vi "pharmaBot_v0.019.vi"() -> ()   [LabVIEW 2015] (continued)
    tunnel: [w833] -> w396
    tunnel: w394 -> [w832]
    tunnel: w392 -> [_]
    tunnel: w270 -> [w826]
    tunnel: w272 -> [w825]
    tunnel: w378 -> [w824]
    tunnel: w338 -> [w823]
    shift-right: [w784] -> _
    shift-left: user_message_v6."Initializing..." ("P1 state") -> [w783]
    tunnel: w337 -> [w781]
    tunnel: w245 -> [w780]
    tunnel: w246 -> [w779]
    tunnel: [w778] -> _
    stop <- w835 stop-if-true
    # "Jumper Positions"
    # "Pipette 1 state"
    # "Add the reserved cell index from each manip when checking to see if a cell index can be added back to the queue."
    # "transform cluster + actuator"
    # "positions"
    # "Update the patched cell value visible to the user in the config menu when adding cells back into the array"
    # "If the next or previous button exceeds the index size of the patched cell indicies variable, then disable the corresponding button."
    # "Constantly check to see if there are any \ncells that have been marked as \"patched\""
    n667 = local read "Calibration Protocol"() -> (w787:T7)
    n668 = Wait (ms)(milliseconds to wait=u32 100) -> ()  [unwired: 1 out]
    n669 = local read "P1 state"() -> (w782:T11)
    n670 = local read "Patched Cell Indicies"() -> (w812:i32[])
    n671 = local read "Patched Cell Index"() -> (w811:dbl)
    n672 = local read "cells (image px)"() -> (w822:dbl[][])
    n673 = local read "Patched Cell Index"() -> (w807:dbl)
    n674 = local read "Calibrate:"() -> (w829:T8)
    n675 = local read "current cell 1"() -> (w797:i32)
    n676 = local read "unpatched cell indices"() -> (w798:i32[])
    n677 = Array Size(array=w812) -> (size(s)=w800:i32)
    n678 = Array Size(array=w822) -> (size(s)=w819:i32[])
    n679 = Increment(x=w811) -> (x+1=w810:dbl)
    n680 = Decrement(x=w807) -> (x-1=w805:dbl)
    n681 = Decrement(x=w800) -> (x-1=w799:i32)
    n682 = Index Array(array=w819, index=1) -> (element=w814:i32)
    n683 = Search 1D Array(1D array=w798, element=w797) -> (index of element=w796:i32)  [unwired: 1 in]
    n684 = Greater?(x=w810, y=w799) -> (0:w808:bool)
    n685 = Less?(x=w805, y=0.0) -> (x < y?=w806:bool)
    n686 = case shown="True" w808 {
      tunnel: [T56."Enabled" ("Disabled") T56."Disabled and Grayed Out" ("Disabled")] -> w809
      frame False {
      }
      frame True {
      }
    }
    n687 = case shown="True" w806 {
      tunnel: [T56."Enabled" ("Disabled") T56."Disabled and Grayed Out" ("Disabled")] -> w803
      frame False {
      }
      frame True {
      }
    }
    n688 = Less?(x=w796, y=0) -> (x < y?=w794:bool)
    n689 = case shown="\"manipulator 1\", Default" w829 {
      tunnel: [w854 w856 w858 w860] -> w776
      tunnel: ["Manip 1:" "Manip 2:" "Manip 3:" "Manip 4:"] -> w775
      frame "manipulator 1", Default {
        n690 = local read "current manip 1 pos (steps)"() -> (w854:i32[])
      }
      frame "manipulator 2" {
        n691 = local read "current manip 2 pos (steps)"() -> (w856:i32[])
      }
      frame "manipulator 3" {
        n692 = local read "current manip 3 pos (steps)"() -> (w858:i32[])
      }
      frame "manipulator 4" {
        n693 = local read "current manip 4 pos (steps)"() -> (w860:i32[])
      }
    }
    n694 = for {
      N: w814 -> [_]
      shift-right: [w850] -> w815
      shift-left: i32[] [] ("manip 1 cell indices 2") -> [w852]
      i -> [w851]
      n695 = Build Array (concatenate)(w852, w851) -> (w850:i32[])
    }
    n696 = case shown="True" w794 {
      tunnel: w798 -> [w840 w843]
      tunnel: [w840 w842] -> w793
      tunnel: w797 -> [_ w841]
      frame False {
      }
      frame True {
        n697 = Build Array (concatenate)(w843, w841) -> (w842:i32[])
      }
    }
    n698 = local read "current cell 2"() -> (w792:i32)
    n699 = Search 1D Array(1D array=w793, element=w792) -> (index of element=w791:i32)  [unwired: 1 in]
    n700 = Less?(x=w791, y=0) -> (x < y?=w789:bool)
    n701 = case shown="True" w789 {
      tunnel: w793 -> [w836 w839]
      tunnel: [w836 w838] -> w774
      tunnel: w792 -> [_ w837]
      frame False {
      }
      frame True {
        n702 = Build Array (concatenate)(w839, w837) -> (w838:i32[])
      }
    }
    n703 = case shown="\"Finish\"" w787 {
      tunnel: [w863 w878 w894 w919 w972 w980 w992 w1052 w1095 w1106 w1125 w1228 w1313 w1319 w1350] -> w830
      tunnel: w787 -> [w863 w877 w893 w920 w971 w979 w991 w1051 w1094 w1105 w1125 w1227 w1312 w1319 w1349]
      tunnel: [_ _ w891 _ _ _ _ _ w1093 w1104 _ _ _ _ _] -> _
      tunnel: [_ _ w891 _ _ _ _ _ w1093 w1104 _ _ _ _ _] -> _
      tunnel: [_ TRUE ("Visible") w891 w909 w969 w977 w990 w1050 w1093 w1104 _ w1225 TRUE ("Visible") _ TRUE ("Visible")] -> w827
      tunnel: [_ _ w891 w909 w969 w977 w990 w1050 w1093 w1104 _ w1225 _ _ _] -> w828
      tunnel: w826 -> [_ _ _ _ _ _ w988 w1046 w1090 w1101 _ w1222 _ _ _]
      tunnel: w825 -> [_ _ w890 w913 _ _ w987 w1044 w1088 w1099 _ w1220 _ _ _]
      tunnel: w824 -> [_ _ _ _ _ _ w986 w1048 _ _ _ _ _ _ _]
      tunnel: w823 -> [_ _ _ _ _ _ w985 w1047 _ _ _ _ _ _ _]
      tunnel: w774 -> [_ _ _ _ _ _ _ _ _ _ _ _ _ _ w1348]
      tunnel: w814 -> [_ _ _ _ _ _ _ _ _ _ _ _ _ _ w1347]
      tunnel: [w862 w874 w889 w908 w968 w976 w984 w1045 w1089 w1100 w1124 w1221 w1307 w1316 w1339] -> w784
      tunnel: w783 -> [w862 w874 w889 w908 w968 w976 w984 w1045 w1089 w1100 w1124 w1221 w1307 w1318 w1339]
      tunnel: w782 -> [_ _ _ _ _ _ _ _ _ _ _ _ _ w1316 _]
      tunnel: w776 -> [_ _ _ _ _ _ _ _ _ _ w1122 _ _ _ _]
      tunnel: w781 -> [_ _ _ _ _ _ _ _ _ _ w1121 _ _ _ _]
      tunnel: w780 -> [_ _ _ _ _ _ _ _ _ _ w1117 _ _ _ _]
      tunnel: w779 -> [_ _ _ _ _ _ _ _ _ _ w1112 _ _ _ _]
      tunnel: [_ _ _ _ _ _ _ _ _ _ w1114 _ _ _ _] -> w778
      frame "Init", Default {
        n704 = local read "How Many Manipulators?"() -> (w861:enum16{"1", "2", "3", "4"})
        n705 = case shown="\"1\", Default" w861 {
          tunnel: [w868 TRUE ("Visible") w872 w873] -> w866
          tunnel: [w868 w869 w872 w873] -> w865
          tunnel: [w868 w869 FALSE ("Visible") w873] -> w864
          frame "1", Default {
            w868 = FALSE ("Visible")
          }
          frame "2" {
            w869 = FALSE ("Visible")
          }
          frame "3" {
            w872 = TRUE ("Visible")
          }
          frame "4" {
            w873 = TRUE ("Visible")
          }
        }
        n706 = local write "which action on cam"(T6."none" ("which action on cam")) -> ()
        n707 = property on="Manip 2 Calibrated" class="Bool (strict)"("Visible"=w866) -> ()  [unwired: 2 in, 2 out]
        n708 = property on="Manip 3 Calibrated" class="Bool (strict)"("Visible"=w865) -> ()  [unwired: 2 in, 2 out]
        n709 = property on="Manip 4 Calibrated" class="Bool (strict)"("Visible"=w864) -> ()  [unwired: 2 in, 2 out]
      }
      frame "Select Manip" {
        n710 = local read "Accept Button"() -> (w879:bool)
        n711 = local write "which action on cam"(T6."Move pipette" ("which action on cam")) -> ()
        n712 = case shown="True" w879 {
          tunnel: [w880 w886] -> w878
          tunnel: w877 -> [w880 _]
          frame False {
          }
          frame True {
            n713 = invoke on="Accept Button" class="Bool (strict)" method="Reinit To Default"() -> ()  [unwired: 3 in, 3 out]
            n714 = local read "Stage Shift (steps)"() -> (w885:dbl)
            n715 = local read "Stage zeroed?"() -> (w888:bool)
            n716 = Negate(x=w885) -> (-x=w883:dbl)
            n717 = Divide(x=w883, y=10.0) -> (x/y=w882:dbl)
            n718 = Select(t=T57."Find Pipette" ("Calibration Protocol"), s=w888, f=T57."Set Stage" ("Calibration Protocol")) -> (s? t:f=w886:T57)
            n719 = property on="Next Stage and Pipette Z Location" class="Slide (strict)"("Scale.Maximum"=w882) -> ()  [unwired: 2 in, 2 out]
          }
        }
      }
      frame "Set Stage" {
        w891 = TRUE ("Visible")
        n720 = local read "Accept Button"() -> (w895:bool)
        n721 = local write "which action on cam"(T6."Move pipette" ("which action on cam")) -> ()
        n722 = case shown="True" w895 {
          tunnel: [w896 T57."Find Pipette" ("Calibration Protocol")] -> w894
          tunnel: w893 -> [w896 _]
          tunnel: w890 -> [_ w902]
          frame False {
          }
          frame True {
            w901 = 0.0 ("element")
            # "the stage has been zeroed:\nmove the stage up for nxt pipette"
            # "Once the user has zeroed the stage, retract the stage XX steps automatically."
            n723 = invoke on="Accept Button" class="Bool (strict)" method="Reinit To Default"() -> ()  [unwired: 3 in, 3 out]
            n724 = Unbundle By Name(w902) -> ("s"=w905:refnum<vi>)
            n725 = local read "Stage Shift (steps)"() -> (w899:dbl)
            n726 = property class="Clust (strict)"(reference=w905) -> ("Value"=w906:T25)  [unwired: 1 in, 2 out]
            n727 = Multiply(x=w899, y=-7.53) -> (x*y=w898:dbl)
            n728 = Unbundle By Name(w906) -> ("actuator"=w903:T26)
            n729 = Build Array(w901, w901, w898) -> (w904:dbl[])
            n730 = call "moveTo_abs_XYZ.vi"("XYZ location (steps)"=w904, "Actuator cluster in"=w903) -> ()  [unwired: 8 in, 2 out]
          }
        }
      }
      frame "Find Pipette" {
        w909 = TRUE ("Visible")
        n731 = local read "Calibrate:"() -> (w917:T8)
        n732 = case shown="\"manipulator 3\"" w917 {
          tunnel: [w945 w947 w949 w951] -> w916
          tunnel: w913 -> [w944 w946 w948 w950]
          frame "manipulator 1", Default {
            n733 = Unbundle By Name(w944) -> ("manip 1"=w945:refnum<vi>)
          }
          frame "manipulator 2" {
            n734 = Unbundle By Name(w946) -> ("manip 2"=w947:refnum<vi>)
          }
          frame "manipulator 3" {
            n735 = Unbundle By Name(w948) -> ("manip 3"=w949:refnum<vi>)
          }
          frame "manipulator 4" {
            n736 = Unbundle By Name(w950) -> ("manip 4"=w951:refnum<vi>)
          }
        }
        n737 = property class="Clust (strict)"(reference=w916) -> ("Value"=w915:T25)  [unwired: 1 in, 2 out]
        n738 = local read "Pipette is in Focus?"() -> (w911:bool)
        n739 = case shown="False" w911 {
          tunnel: [T56."Enabled" ("Disabled") T56."Disabled and Grayed Out" ("Disabled")] -> w912
          tunnel: [w931 w933] -> w910
          tunnel: [w931 w933] -> w907
          frame False {
            w931 = T56."Disabled and Grayed Out" ("Disabled")
            # "After the pipette is moved out of focus"
          }
          frame True {
            w933 = T56."Enabled" ("Disabled")
            w938 = 2 ("index")
            # "compare \"z\""
            # "While the pipette is in focus..."
            n740 = local read "Current Manip Focus Coords."() -> (w939:i32[])
            n741 = local read "Current Manipulator Position"() -> (w941:i32[])
            n742 = Index Array(array=w941, index=w938) -> (element=w940:i32)
            n743 = Index Array(array=w939, index=w938) -> (element=w937:i32)
            n744 = Subtract(x=w940, y=w937) -> (x-y=w942:i32)
            n745 = Absolute Value(x=w942) -> (abs(x)=w936:i32)
            n746 = Less Or Equal?(x=w936, y="Z focus range for pipette") -> (x <= y?=w934:bool)
            n747 = local write "Pipette is in Focus?"(w934) -> ()
          }
        }
        n748 = local write "which action on cam"(T6."Move pipette" ("which action on cam")) -> ()
        n749 = Unbundle By Name(w915) -> ("actuator"=w914:T26)
        n750 = local read "Accept Button"() -> (w921:bool)
        n751 = case shown="True" w921 {
          tunnel: w920 -> [w952 _]
          tunnel: [w952 T57."Set Safe" ("Calibration Protocol")] -> w919
          tunnel: w914 -> [_ w959]
          frame False {
          }
          frame True {
            # "+ is towards cells!"
            # "After the user has found the pipette and set it's zero, return the pipette to the safe space"
            n752 = local read "step distance (steps) safe space"() -> (w953:dbl)
            n753 = invoke on="Accept Button" class="Bool (strict)" method="Reinit To Default"() -> ()  [unwired: 3 in, 3 out]
            n754 = call "set step.vi"("step distance (steps)"=w953, "actuator in"=w959) -> ("error out"=w962:errorcluster, "actuator out"=w960:T26)  [unwired: 8 in]
            n755 = call "take step.vi"("approach?"=TRUE, "motion"=scope_motion."fast", "error in"=w962, "actuator in"=w960) -> ("error out"=w966:errorcluster, "actuator out"=w965:T26)  [unwired: 6 in]
            n756 = local read "Stage Shift (steps)"() -> (w958:dbl)
            n757 = call "reset manipulator.vi"("error in"=w966, "approach? (T = on)"=FALSE, "motion"=scope_motion."fast", "manip in"=w965) -> ()  [unwired: 6 in, 2 out]
            n758 = Negate(x=w958) -> (-x=w956:dbl)
            n759 = Divide(x=w956, y=10.0) -> (x/y=w955:dbl)
            n760 = property on="Next Stage and Pipette Z Location" class="Slide (strict)"("Scale.Maximum"=w955) -> ()  [unwired: 2 in, 2 out]
          }
        }
        n761 = property on="Zero Pipette 1" class="Bool (strict)"("DisabledEnum"=w907) -> ()  [unwired: 2 in, 2 out]
        n762 = property on="Pipette is in Focus" class="Bool (strict)"("DisabledEnum"=w912) -> ()  [unwired: 2 in, 2 out]
        n763 = property on="Move Stage and Pipette Down" class="Bool (strict)"("DisabledEnum"=w910) -> ()  [unwired: 2 in, 2 out]
        n764 = property on="Zero Pipette 3" class="Bool (strict)"("DisabledEnum"=w907) -> ()  [unwired: 2 in, 2 out]
        n765 = disable-structure shown="Disabled" {
          frame Disabled {
            # "enable the \"zero pipette\" button once the stage is near 0"
            n766 = local read "Z focus range for pipette"() -> (w926:i32)
            n767 = local read "current stage pos (steps)"() -> (w930:i32[])
            n768 = Index Array(array=w930, index=2) -> (element=w928:i32)
            n769 = Absolute Value(x=w928) -> (abs(x)=w927:i32)
            n770 = Less Or Equal?(x=w927, y=w926) -> (x <= y?=w925:bool)
            n771 = Select(t=T56."Enabled" ("Disabled"), s=w925, f=T56."Disabled and Grayed Out" ("Disabled")) -> (s? t:f=w923:T56)
            n772 = property on="Zero Pipette 1" class="Bool (strict)"("DisabledEnum"=w923) -> ()  [unwired: 2 in, 2 out]
          }
          frame Enabled {
          }
        }
      }
      frame "Set Safe" {
        w969 = TRUE ("Visible")
        n773 = local read "Accept Button"() -> (w973:bool)
        n774 = case shown="True" w973 {
          tunnel: [w974 T57."Set LAB" ("Calibration Protocol")] -> w972
          tunnel: w971 -> [w974 _]
          frame False {
          }
          frame True {
            n775 = invoke on="Accept Button" class="Bool (strict)" method="Reinit To Default"() -> ()  [unwired: 3 in, 3 out]
          }
        }
        n776 = local write "which action on cam"(T6."Move pipette" ("which action on cam")) -> ()
      }
      frame "Set LAB" {
        w977 = TRUE ("Visible")
        n777 = local read "Accept Button"() -> (w981:bool)
        n778 = case shown="True" w981 {
          tunnel: [w982 T57."Set Clean" ("Calibration Protocol")] -> w980
          tunnel: w979 -> [w982 _]
          frame False {
          }
          frame True {
            n779 = invoke on="Accept Button" class="Bool (strict)" method="Reinit To Default"() -> ()  [unwired: 3 in, 3 out]
          }
        }
        n780 = local write "which action on cam"(T6."Move pipette" ("which action on cam")) -> ()
      }
      frame "Set Clean" {
        w990 = TRUE ("Visible")
        # "manip 2"
        # "Manip 1"
        n781 = local read "Accept Button"() -> (w993:bool)
        n782 = case shown="True" w993 {
          tunnel: [w994 T57."Set Wash" ("Calibration Protocol")] -> w992
          tunnel: w991 -> [w994 _]
          tunnel: w988 -> [_ w1000]
          tunnel: w987 -> [_ w999]
          tunnel: w986 -> [_ w1004]
          tunnel: w985 -> [_ w1002]
          frame False {
          }
          frame True {
            w997 = TRUE ("blocking?")
            n783 = local read "Calibrate:"() -> (w998:T8)
            n784 = case shown="\"manipulator 2\"" w998 {
              tunnel: w1004 -> [w1022 _ _ _]
              tunnel: [w1017 w1036 _ _] -> w1003
              tunnel: w1002 -> [_ w1043 _ _]
              tunnel: [w1012 w1027 _ _] -> w996
              frame "manipulator 1", Default {
                # "Y"
                # "X"
                n785 = local read "loc above baths 1"() -> (w1021:i32[])
                n786 = local read "Manip 1 Distance [mm]"() -> (w1006:dbl)
                n787 = local read "Manip 1 Angle [deg]"() -> (w1005:dbl)
                n788 = call "get_XYZ.vi"("Actuator cluster in"=w1022) -> ("X pos (steps)"=w1023:i32, "Y pos (steps)"=w1024:i32)  [unwired: 10 in, 3 out]
                n789 = expression code="(x/180.0)*pi" "degrees to radians"(w1005) -> (w1016:dbl)
                n790 = Multiply(x=w1006, y=10000.0) -> (x*y=w1009:dbl)
                n791 = Array Subset(array=w1021, index=2, length=1) -> (w1018:i32[])
                n792 = Build Array (concatenate)(w1023, w1024, w1018) -> (w1017:i32[])
                n793 = Cosine(x=w1016) -> (cos(x)=w1015:dbl)
                n794 = Sine(x=w1016) -> (sin(x)=w1014:dbl)
                n795 = Multiply(x=w1009, y=w1014) -> (x*y=w1008:dbl)
                n796 = Multiply(x=w1009, y=w1015) -> (x*y=w1013:dbl)
                n797 = Negate(x=w1008) -> (-x=w1007:dbl)
                n798 = Build Array(w1013, w1007, 0.0 ("element")) -> (w1012:dbl[])
              }
              frame "manipulator 2" {
                n799 = local read "Manip 2 Angle [deg]"() -> (w1025:dbl)
                n800 = local read "Manip 2 Distance [mm]"() -> (w1026:dbl)
                n801 = local read "loc above baths 2"() -> (w1038:i32[])
                n802 = call "get_XYZ.vi"("Actuator cluster in"=w1043) -> ("X pos (steps)"=w1042:i32, "Y pos (steps)"=w1041:i32)  [unwired: 10 in, 3 out]
                n803 = expression code="(x/180.0)*pi" "degrees to radians"(w1025) -> (w1035:dbl)
                n804 = Multiply(x=w1026, y=10000.0) -> (x*y=w1032:dbl)
                n805 = Array Subset(array=w1038, index=2, length=1) -> (w1037:i32[])
                n806 = Build Array (concatenate)(w1042, w1041, w1037) -> (w1036:i32[])
                n807 = Cosine(x=w1035) -> (cos(x)=w1033:dbl)
                n808 = Sine(x=w1035) -> (sin(x)=w1031:dbl)
                n809 = Multiply(x=w1032, y=w1033) -> (x*y=w1030:dbl)
                n810 = Multiply(x=w1032, y=w1031) -> (x*y=w1029:dbl)
                n811 = Build Array(w1030, w1029, 0.0 ("element")) -> (w1027:dbl[])
              }
              frame "manipulator 3" {
              }
              frame "manipulator 4" {
              }
            }
            n812 = invoke on="Accept Button" class="Bool (strict)" method="Reinit To Default"() -> ()  [unwired: 3 in, 3 out]
            n813 = call "move manipulator abs xyz.vi"("blocking?"=w997, "which manipulator"=w998, "transform cluster + actuator"=w999, "positions"=w1000, "location (steps)"=w1003) -> ("error out"=w1001:errorcluster)  [unwired: 6 in]
            n814 = call "move manipulator rel.vi"("blocking?"=w997, "which manipulator"=w998, "error in (no error)"=w1001, "transform cluster + actuator"=w999, "positions"=w1000, "location (steps)"=w996) -> ()  [unwired: 5 in, 1 out]
          }
        }
        n815 = local write "which action on cam"(T6."Move pipette" ("which action on cam")) -> ()
      }
      frame "Set Wash" {
        w1050 = TRUE ("Visible")
        n816 = local read "Accept Button"() -> (w1053:bool)
        n817 = case shown="True" w1053 {
          tunnel: [w1054 T57."Reset 0s" ("Calibration Protocol")] -> w1052
          tunnel: w1051 -> [w1054 _]
          tunnel: w1048 -> [_ w1067]
          tunnel: w1047 -> [_ w1066]
          tunnel: w1046 -> [_ w1061]
          tunnel: w1044 -> [_ w1060]
          tunnel: w1044 -> [_ w1059]
          frame False {
          }
          frame True {
            w1062 = TRUE ("blocking?")
            n818 = local read "Calibrate:"() -> (w1063:T8)
            n819 = case shown="\"manipulator 1\", Default" w1063 {
              tunnel: w1067 -> [w1077 _ _ _]
              tunnel: w1066 -> [_ w1087 _ _]
              tunnel: [w1068 w1080 _ _] -> w1065
              tunnel: w1059 -> [w1076 w1079 _ _]
              tunnel: [w1075 w1078 _ _] -> w1057
              frame "manipulator 1", Default {
                n820 = local read "loc above baths 1"() -> (w1072:i32[])
                n821 = call "get_XYZ.vi"("Actuator cluster in"=w1077) -> ("X pos (steps)"=w1074:i32, "Y pos (steps)"=w1073:i32)  [unwired: 10 in, 3 out]
                n822 = Unbundle By Name(w1076) -> ("manip 1"=w1075:refnum<vi>)
                n823 = Array Subset(array=w1072, index=2, length=1) -> (w1069:i32[])
                n824 = Build Array (concatenate)(w1074, w1073, w1069) -> (w1068:i32[])
              }
              frame "manipulator 2" {
                n825 = local read "loc above baths 2"() -> (w1084:i32[])
                n826 = Unbundle By Name(w1079) -> ("manip 2"=w1078:refnum<vi>)
                n827 = call "get_XYZ.vi"("Actuator cluster in"=w1087) -> ("X pos (steps)"=w1086:i32, "Y pos (steps)"=w1085:i32)  [unwired: 10 in, 3 out]
                n828 = Array Subset(array=w1084, index=2, length=1) -> (w1081:i32[])
                n829 = Build Array (concatenate)(w1086, w1085, w1081) -> (w1080:i32[])
              }
              frame "manipulator 3" {
              }
              frame "manipulator 4" {
              }
            }
            n830 = property class="Clust (strict)"(reference=w1057) -> ("Value"=w1058:T25)  [unwired: 1 in, 2 out]
            n831 = invoke on="Accept Button" class="Bool (strict)" method="Reinit To Default"() -> ()  [unwired: 3 in, 3 out]
            n832 = Unbundle By Name(w1058) -> ("safe space (steps)"=w1056:i32[])
            n833 = call "move manipulator abs xyz.vi"("blocking?"=w1062, "which manipulator"=w1063, "transform cluster + actuator"=w1060, "positions"=w1061, "location (steps)"=w1065) -> ("error out"=w1064:errorcluster)  [unwired: 6 in]
            n834 = call "move manipulator abs xyz.vi"("blocking?"=w1062, "which manipulator"=w1063, "error in (no error)"=w1064, "transform cluster + actuator"=w1060, "positions"=w1061, "location (steps)"=w1056) -> ()  [unwired: 5 in, 1 out]
          }
        }
        n835 = local write "which action on cam"(T6."Move pipette" ("which action on cam")) -> ()
      }
      frame "Reset 0s" {
        w1093 = TRUE ("Visible")
        n836 = local read "Accept Button"() -> (w1096:bool)
        n837 = property on="Accept Button" class="Bool (strict)"("DisabledEnum"=T56."Enabled" ("Disabled")) -> ()  [unwired: 2 in, 2 out]
        n838 = case shown="True" w1096 {
          tunnel: [w1097 T57."Pipette Template" ("Calibration Protocol")] -> w1095
          tunnel: w1094 -> [w1097 _]
          tunnel: w1090 -> [_ _]
          tunnel: w1088 -> [_ _]
          frame False {
          }
          frame True {
            n839 = invoke on="Accept Button" class="Bool (strict)" method="Reinit To Default"() -> ()  [unwired: 3 in, 3 out]
          }
        }
        n840 = local write "which action on cam"(T6."Move pipette" ("which action on cam")) -> ()
      }
      frame "Change pipette" {
        w1104 = TRUE ("Visible")
        n841 = local read "Accept Button"() -> (w1107:bool)
        n842 = property on="Accept Button" class="Bool (strict)"("DisabledEnum"=T56."Enabled" ("Disabled")) -> ()  [unwired: 2 in, 2 out]
        n843 = case shown="True" w1107 {
          tunnel: [w1108 T57."Pipette Template" ("Calibration Protocol")] -> w1106
          tunnel: w1105 -> [w1108 _]
          tunnel: w1101 -> [_ _]
          tunnel: w1099 -> [_ _]
          frame False {
          }
          frame True {
            n844 = invoke on="Accept Button" class="Bool (strict)" method="Reinit To Default"() -> ()  [unwired: 3 in, 3 out]
          }
        }
        n845 = local write "which action on cam"(T6."Move pipette" ("which action on cam")) -> ()
      }
      frame "Set Jumper" {
        n846 = local read "Which Jumper Position to Set?"() -> (w1119:T9)
        n847 = local read "Manip Jump"() -> (w1110:bool)
        n848 = property on="Which Manip Jumper Position?" class="Enum (strict)"("Visible"=w1110) -> ()  [unwired: 2 in, 2 out]
        n849 = local read "go to jumper position"() -> (w1118:bool)
        n850 = local read "Choose Position"() -> (w1114:bool)
        n851 = case shown="\"Jumper Safe Position\"" w1119 {
          tunnel: [FALSE FALSE FALSE FALSE FALSE TRUE TRUE TRUE TRUE TRUE TRUE TRUE TRUE] -> w1115
          tunnel: [TRUE TRUE TRUE TRUE TRUE TRUE TRUE TRUE TRUE TRUE TRUE TRUE TRUE] -> w1123
          tunnel: w1114 -> [w1141 w1148 w1154 w1160 w1166 w1172 w1178 w1184 w1190 w1196 w1202 w1208 w1214]
          tunnel: w1122 -> [w1142 w1149 w1155 w1161 w1167 w1173 w1179 w1185 w1191 w1197 w1203 w1209 w1215]
          tunnel: w1121 -> [_ _ _ _ _ _ _ _ _ _ _ _ _]
          tunnel: [_ errorcluster {"status"=FALSE, "code"=0, "source"=""} ("error in (no error)") _ _ _ _ _ _ _ _ _ _ _] -> w1113
          frame "Jumper Safe Position" {
            n852 = case shown="True" w1141 {
              tunnel: w1141 -> [_ w1146]
              tunnel: w1142 -> [_ w1145]
              frame False {
              }
              frame True {
                n853 = local write "Jumper Safe"(w1146) -> ()
                n854 = local write "Jumper Safe Position"(w1145) -> ()
              }
            }
          }
          frame "Experiment Safe Position" {
            n855 = case shown="True" w1148 {
              tunnel: w1148 -> [_ w1153]
              tunnel: w1149 -> [_ w1152]
              frame False {
              }
              frame True {
                n856 = local write "Experiment Safe"(w1153) -> ()
                n857 = local write "Experiment Safe Position"(w1152) -> ()
              }
            }
          }
          frame "Jumper Position A" {
            n858 = case shown="True" w1154 {
              tunnel: w1154 -> [_ w1159]
              tunnel: w1155 -> [_ w1158]
              frame False {
              }
              frame True {
                n859 = local write "Pos A"(w1159) -> ()
                n860 = local write "Jumper Position A"(w1158) -> ()
              }
            }
          }
          frame "Jumper Position B" {
            n861 = case shown="True" w1160 {
              tunnel: w1160 -> [_ w1165]
              tunnel: w1161 -> [_ w1164]
              frame False {
              }
              frame True {
                n862 = local write "Pos B"(w1165) -> ()
                n863 = local write "Jumper Position B"(w1164) -> ()
              }
            }
          }
          frame "Jumper Position C" {
            n864 = case shown="True" w1166 {
              tunnel: w1167 -> [_ w1171]
              tunnel: w1166 -> [_ w1170]
              frame False {
              }
              frame True {
                n865 = local write "Pos C"(w1170) -> ()
                n866 = local write "Jumper Position C"(w1171) -> ()
              }
            }
          }
          frame "Jumper Position o-A" {
            n867 = case shown="True" w1172 {
              tunnel: w1172 -> [_ w1177]
              tunnel: w1173 -> [_ w1176]
              frame False {
              }
              frame True {
                n868 = local write "Jump Pos o-A"(w1177) -> ()
                n869 = local write "Jumper Position o-A"(w1176) -> ()
              }
            }
          }
          frame "Jumper Position A-o" {
            n870 = case shown="True" w1178 {
              tunnel: w1178 -> [_ w1183]
              tunnel: w1179 -> [_ w1182]
              frame False {
              }
              frame True {
                n871 = local write "Jump Pos A-o"(w1183) -> ()
                n872 = local write "Jumper Position A-o"(w1182) -> ()
              }
            }
          }
          frame "Jumper Position A-B" {
            n873 = case shown="True" w1184 {
              tunnel: w1184 -> [_ w1189]
              tunnel: w1185 -> [_ w1188]
              frame False {
              }
              frame True {
                n874 = local write "Jump Pos A-B"(w1189) -> ()
                n875 = local write "Jumper Position A-B"(w1188) -> ()
              }
            }
          }
          frame "Jumper Position B-A" {
            n876 = case shown="True" w1190 {
              tunnel: w1190 -> [_ w1195]
              tunnel: w1191 -> [_ w1194]
              frame False {
              }
              frame True {
                n877 = local write "Jump Pos B-A"(w1195) -> ()
                n878 = local write "Jumper Position B-A"(w1194) -> ()
              }
            }
          }
          frame "Jumper Position B-C" {
            n879 = case shown="True" w1196 {
              tunnel: w1196 -> [_ w1201]
              tunnel: w1197 -> [_ w1200]
              frame False {
              }
              frame True {
                n880 = local write "Jump Pos B-C"(w1201) -> ()
                n881 = local write "Jumper Position B-C"(w1200) -> ()
              }
            }
          }
          frame "Jumper Position C-B" {
            n882 = case shown="True" w1202 {
              tunnel: w1202 -> [_ w1207]
              tunnel: w1203 -> [_ w1206]
              frame False {
              }
              frame True {
                n883 = local write "Jump Pos C-B"(w1207) -> ()
                n884 = local write "Jumper Position C-B"(w1206) -> ()
              }
            }
          }
          frame "Jumper Position C-o" {
            n885 = case shown="True" w1208 {
              tunnel: w1208 -> [_ w1213]
              tunnel: w1209 -> [_ w1212]
              frame False {
              }
              frame True {
                n886 = local write "Jump Pos C-o"(w1213) -> ()
                n887 = local write "Jumper Position C-o"(w1212) -> ()
              }
            }
          }
          frame "Jumper Position o-C" {
            n888 = case shown="True" w1214 {
              tunnel: w1214 -> [_ w1219]
              tunnel: w1215 -> [_ w1218]
              frame False {
              }
              frame True {
                n889 = local write "Jump Pos o-C"(w1219) -> ()
                n890 = local write "Jumper Position o-C"(w1218) -> ()
              }
            }
          }
        }
        n891 = case shown="True" w1118 {
          tunnel: w1117 -> [_ w1140]
          tunnel: w1112 -> [_ _]
          tunnel: w1119 -> [_ w1139]
          tunnel: T8."manipulator 1" ("which manipulator") -> [_ w1138]
          frame False {
          }
          frame True {
            n892 = call "moveToJumperPosition-v02.vi"("which manipulator"=w1138, "Which Jumper Position to move to?"=w1139, "setStatus?"=FALSE, "common cluster"=w1140) -> ("error out"=w1137:errorcluster)  [unwired: 10 in, 1 out]
            n893 = call "Time Delay3"("error in (no error)"=w1137) -> ()  [unwired: 10 in, 1 out]
          }
        }
        n894 = local read "memtest 1"() -> (w1116:waveform(dbl))
        n895 = local write "memtestJumperMonitor"(w1116) -> ()
        n896 = Or(x=w1115, y=w1110) -> (x .or. y?=w1111:bool)
        n897 = property on="Jump Trigger" class="Bool (strict)"("Visible"=w1111) -> ()  [unwired: 2 in, 2 out]
        n898 = case shown="True" w1114 {
          tunnel: w1113 -> [_ w1126]
          frame False {
          }
          frame True {
            n899 = flat-sequence {
              tunnel: w1127 -> [w1132]
              tunnel: [w1131] -> w1128
              tunnel: w1126 -> [w1129]
              tunnel: w1128 -> [w1134]
              frame #0 {
                n900 = property class="Bool (strict)"(reference=w1132, error in=w1129, "Val(Sgnl)"=TRUE ("Value")) -> (reference out=w1131:refnum<vi>)  [unwired: 1 out]
              }
              frame #1 {
                n901 = property class="Bool (strict)"(reference=w1134, "Val(Sgnl)"=FALSE ("Value")) -> ()  [unwired: 1 in, 2 out]
              }
              frame #2 {
                n902 = local write "Choose Position"(FALSE ("Choose Position")) -> ()
              }
            }
            n903 = control-ref of="save locations 2"() -> (w1127:refnum<vi>)
          }
        }
        n904 = property on="jumptestMonitor" class="WFGraph (strict)"("Visible"=w1111) -> ()  [unwired: 2 in, 2 out]
        n905 = property on="memtestJumperMonitor" class="WFGraph (strict)"("Visible"=w1123) -> ()  [unwired: 2 in, 2 out]
      }
      frame "Pipette Template" {
        w1225 = TRUE ("Visible")
        n906 = local read "Accept Button"() -> (w1226:bool)
        n907 = case shown="True" w1226 {
          tunnel: [w1229 w1230] -> w1228
          tunnel: w1227 -> [w1229 _]
          tunnel: w1222 -> [_ w1234]
          tunnel: w1220 -> [_ w1231]
          tunnel: w1220 -> [_ w1233]
          frame False {
          }
          frame True {
            # "determine if you need to calibrate another manip"
            # "set currently selected manip to calibrated state"
            # "When done with the pipette template..."
            n908 = local read "Calibrate:"() -> (w1235:T8)
            n909 = local read "How Many Manipulators?"() -> (w1241:enum16{"1", "2", "3", "4"})
            n910 = case shown="\"4\"" w1241 {
              tunnel: [w1251 w1252 w1258 w1270] -> w1240
              tunnel: w1235 -> [_ w1253 w1259 w1271]
              frame "1", Default {
                (unwired) 1.0
                n911 = local read "Manip 1 Calibrated"() -> (w1251:bool)
              }
              frame "2" {
                n912 = case shown="\"manipulator 1\", Default" w1253 {
                  tunnel: [w1254 w1255 TRUE ("Manip 1 Calibrated") TRUE ("Manip 1 Calibrated")] -> w1252
                  frame "manipulator 1", Default {
                    n913 = local read "Manip 2 Calibrated"() -> (w1254:bool)
                  }
                  frame "manipulator 2" {
                    n914 = local read "Manip 1 Calibrated"() -> (w1255:bool)
                  }
                  frame "manipulator 3" {
                  }
                  frame "manipulator 4" {
                  }
                }
              }
              frame "3" {
                n915 = case shown="\"manipulator 4\"" w1259 {
                  tunnel: [w1262 w1263 w1268 TRUE] -> w1258
                  frame "manipulator 1", Default {
                    n916 = local read "Manip 3 Calibrated"() -> (w1261:bool)
                    n917 = local read "Manip 2 Calibrated"() -> (w1260:bool)
                    n918 = And(x=w1260, y=w1261) -> (x .and. y?=w1262:bool)
                  }
                  frame "manipulator 2" {
                    n919 = local read "Manip 1 Calibrated"() -> (w1265:bool)
                    n920 = local read "Manip 3 Calibrated"() -> (w1264:bool)
                    n921 = And(x=w1265, y=w1264) -> (x .and. y?=w1263:bool)
                  }
                  frame "manipulator 3" {
                    n922 = local read "Manip 1 Calibrated"() -> (w1267:bool)
                    n923 = local read "Manip 2 Calibrated"() -> (w1266:bool)
                    n924 = And(x=w1267, y=w1266) -> (x .and. y?=w1268:bool)
                  }
                  frame "manipulator 4" {
                  }
                }
              }
              frame "4" {
                n925 = case shown="\"manipulator 1\", Default" w1271 {
                  tunnel: [w1272 w1281 w1286 w1291] -> w1270
                  frame "manipulator 1", Default {
                    n926 = local read "Manip 4 Calibrated"() -> (w1273:bool)
                    n927 = local read "Manip 3 Calibrated"() -> (w1274:bool)
                    n928 = local read "Manip 2 Calibrated"() -> (w1275:bool)
                    n929 = And(x=w1274, y=w1273) -> (x .and. y?=w1276:bool)
                    n930 = And(x=w1275, y=w1276) -> (x .and. y?=w1272:bool)
                  }
                  frame "manipulator 2" {
                    n931 = local read "Manip 1 Calibrated"() -> (w1279:bool)
                    n932 = local read "Manip 3 Calibrated"() -> (w1278:bool)
                    n933 = local read "Manip 4 Calibrated"() -> (w1277:bool)
                    n934 = And(x=w1278, y=w1277) -> (x .and. y?=w1280:bool)
                    n935 = And(x=w1279, y=w1280) -> (x .and. y?=w1281:bool)
                  }
                  frame "manipulator 3" {
                    n936 = local read "Manip 1 Calibrated"() -> (w1284:bool)
                    n937 = local read "Manip 2 Calibrated"() -> (w1283:bool)
                    n938 = local read "Manip 4 Calibrated"() -> (w1282:bool)
                    n939 = And(x=w1283, y=w1282) -> (x .and. y?=w1285:bool)
                    n940 = And(x=w1284, y=w1285) -> (x .and. y?=w1286:bool)
                  }
                  frame "manipulator 4" {
                    n941 = local read "Manip 3 Calibrated"() -> (w1287:bool)
                    n942 = local read "Manip 1 Calibrated"() -> (w1289:bool)
                    n943 = local read "Manip 2 Calibrated"() -> (w1288:bool)
                    n944 = And(x=w1288, y=w1287) -> (x .and. y?=w1290:bool)
                    n945 = And(x=w1289, y=w1290) -> (x .and. y?=w1291:bool)
                  }
                }
              }
            }
            n946 = case shown="\"manipulator 4\"" w1235 {
              tunnel: TRUE ("Visible") -> [w1303 w1304 w1305 w1306]
              frame "manipulator 1", Default {
                n947 = local write "Manip 1 Calibrated"(w1303) -> ()
              }
              frame "manipulator 2" {
                n948 = local write "Manip 2 Calibrated"(w1304) -> ()
              }
              frame "manipulator 3" {
                n949 = local write "Manip 3 Calibrated"(w1305) -> ()
              }
              frame "manipulator 4" {
                n950 = local write "Manip 4 Calibrated"(w1306) -> ()
              }
            }
            n951 = case shown="\"manipulator 4\"" w1235 {
              tunnel: [w1244 w1246 w1248 w1250] -> w1239
              tunnel: w1233 -> [w1243 w1245 w1247 w1249]
              frame "manipulator 1", Default {
                n952 = Unbundle By Name(w1243) -> ("manip 1"=w1244:refnum<vi>)
              }
              frame "manipulator 2" {
                n953 = Unbundle By Name(w1245) -> ("manip 2"=w1246:refnum<vi>)
              }
              frame "manipulator 3" {
                n954 = Unbundle By Name(w1247) -> ("manip 3"=w1248:refnum<vi>)
              }
              frame "manipulator 4" {
                n955 = Unbundle By Name(w1249) -> ("manip 4"=w1250:refnum<vi>)
              }
            }
            n956 = local read "Stage zeroed?"() -> (w1232:bool)
            n957 = property class="Clust (strict)"(reference=w1239) -> ("Value"=w1238:T25)  [unwired: 1 in, 2 out]
            n958 = Unbundle By Name(w1238) -> ("safe space (steps)"=w1237:i32[])
            n959 = case shown="False" w1240 {
              tunnel: w1232 -> [w1294 _]
              tunnel: w1231 -> [w1293 _]
              tunnel: [T57."Select Manip" ("Calibration Protocol") T57."Add Cells" ("Calibration Protocol")] -> w1230
              frame False {
                # "Not done calibrating"
                n960 = case shown="True" w1294 {
                  tunnel: w1293 -> [_ w1295]
                  frame False {
                  }
                  frame True {
                    w1299 = 0.0 ("element")
                    # "the stage has been zeroed:\nmove the stage up for nxt pipette"
                    n961 = Unbundle By Name(w1295) -> ("s"=w1300:refnum<vi>)
                    n962 = local read "Stage Shift (steps)"() -> (w1298:dbl)
                    n963 = property class="Clust (strict)"(reference=w1300) -> ("Value"=w1301:T25)  [unwired: 1 in, 2 out]
                    n964 = Unbundle By Name(w1301) -> ("actuator"=w1296:T26)
                    n965 = Build Array(w1299, w1299, w1298) -> (w1297:dbl[])
                    n966 = call "moveTo_abs_XYZ.vi"("XYZ location (steps)"=w1297, "Actuator cluster in"=w1296) -> ()  [unwired: 8 in, 2 out]
                  }
                }
              }
              frame True {
                # "done calibrating"
              }
            }
            n967 = call "move manipulator abs xyz.vi"("blocking?"=TRUE, "which manipulator"=w1235, "transform cluster + actuator"=w1231, "positions"=w1234, "location (steps)"=w1237) -> ()  [unwired: 6 in, 1 out]
            n968 = invoke on="Accept Button" class="Bool (strict)" method="Reinit To Default"() -> ()  [unwired: 3 in, 3 out]
          }
        }
        n969 = local write "which action on cam"(T6."Pipette template" ("which action on cam")) -> ()
        n970 = property on="Accept Button" class="Bool (strict)"("DisabledEnum"=T56."Enabled" ("Disabled")) -> ()  [unwired: 2 in, 2 out]
      }
      frame "Add Cells" {
        n971 = local read "Accept Button"() -> (w1311:bool)
        n972 = case shown="True" w1311 {
          tunnel: [w1314 T57."Finish" ("Calibration Protocol")] -> w1313
          tunnel: w1312 -> [w1314 _]
          frame False {
          }
          frame True {
            n973 = invoke on="Accept Button" class="Bool (strict)" method="Reinit To Default"() -> ()  [unwired: 3 in, 3 out]
          }
        }
        n974 = local write "which action on cam"(T6."Add cell" ("which action on cam")) -> ()
        n975 = property on="Accept Button" class="Bool (strict)"("DisabledEnum"=T56."Enabled" ("Disabled")) -> ()  [unwired: 2 in, 2 out]
      }
      frame "Finish" {
        n976 = local write "which action on cam"(T6."Move pipette" ("which action on cam")) -> ()
        n977 = Not Equal?(x=w1316, y=w1318) -> (x != y?=w1317:bool)
        n978 = case shown="True" w1317 {
          tunnel: w1316 -> [_ w1321]
          frame False {
            # "If the pipette has NOT changed state"
          }
          frame True {
            # "If the pipette has just changed state..."
            n979 = Equal?(x=w1321, y=user_message_v6."Gigaseal Established..." ("P1 state")) -> (x = y?=w1326:bool)
            n980 = Equal?(x=w1321, y=user_message_v6."reclean" ("P1 state")) -> (x = y?=w1322:bool)
            n981 = Equal?(x=w1321, y=user_message_v6."Starting new attempt..." ("P1 state")) -> (x = y?=w1328:bool)
            n982 = Equal?(x=w1321, y=user_message_v6."Successful breakin!" ("P1 state")) -> (x = y?=w1324:bool)
            n983 = case shown="True" w1322 {
              frame False {
              }
              frame True {
                # "And the new state is starting new attempt..."
                n984 = local read "nAttempts"() -> (w1331:dbl)
                n985 = Decrement(x=w1331) -> (x-1=w1330:dbl)
                n986 = local write "nAttempts"(w1330) -> ()
              }
            }
            n987 = case shown="True" w1328 {
              frame False {
              }
              frame True {
                # "And the new state is starting new attempt..."
                n988 = local read "nAttempts"() -> (w1337:dbl)
                n989 = Increment(x=w1337) -> (x+1=w1336:dbl)
                n990 = local write "nAttempts"(w1336) -> ()
              }
            }
            n991 = case shown="True" w1326 {
              frame False {
              }
              frame True {
                # "and the new state is a gigaseal..."
                n992 = local read "nGS"() -> (w1335:dbl)
                n993 = Increment(x=w1335) -> (x+1=w1334:dbl)
                n994 = local write "nGS"(w1334) -> ()
              }
            }
            n995 = case shown="True" w1324 {
              frame False {
              }
              frame True {
                # "and the new state is successful breakin!..."
                n996 = local read "nWC"() -> (w1333:dbl)
                n997 = Increment(x=w1333) -> (x+1=w1332:dbl)
                n998 = local write "nWC"(w1332) -> ()
              }
            }
          }
        }
      }
      frame "Load Old Cells" {
        # "diable add cell button once all possible cells have been added back"
        # "unpatched cells index + reserved cells"
        # "Compare the cell indicies with those in the unpatched cell indicies variable. Build the missing indicies into a \nnew array and make this into a drop-down (enum) ring to add back to the cell arrays."
        n999 = local read "Accept Button"() -> (w1351:bool)
        n1000 = for {
          N: w1347 -> [_]
          tunnel: w1348 -> [w1359]
          shift-right: [w1354] -> w1338
          shift-left: i32[] [] ("manip 1 cell indices 2") -> [w1355]
          i -> [w1353]
          # "look for what indicies are missing in the \nunpatched cell array. The search function \nreturns index == -1 if the value DOESN'T exist."
          n1001 = Search 1D Array(1D array=w1359, element=w1353) -> (index of element=w1358:i32)  [unwired: 1 in]
          n1002 = Greater Or Equal?(x=w1358, y=0) -> (x >= y?=w1356:bool)
          n1003 = case shown="False" w1356 {
            tunnel: w1355 -> [w1362 w1363]
            tunnel: [w1360 w1363] -> w1354
            tunnel: w1353 -> [w1361 _]
            frame False {
              n1004 = Build Array (concatenate)(w1362, w1361) -> (w1360:i32[])
            }
            frame True {
            }
          }
        }
        n1005 = case shown="True" w1351 {
          tunnel: [w1364 T57."Finish" ("Calibration Protocol")] -> w1350
          tunnel: w1349 -> [w1364 _]
          frame False {
          }
          frame True {
            n1006 = invoke on="Accept Button" class="Bool (strict)" method="Reinit To Default"() -> ()  [unwired: 3 in, 3 out]
          }
        }
        n1007 = Array Size(array=w1338) -> (size(s)=w1345:i32)
        n1008 = Greater?(x=w1345, y=0) -> (0:w1342:bool)
        n1009 = local write "Patched Cell Indicies"(w1338) -> ()
        n1010 = Select(t=T56."Enabled" ("Disabled"), s=w1342, f=T56."Disabled and Grayed Out" ("Disabled")) -> (s? t:f=w1341:T56)
        n1011 = property on="Add this cell index into queue" class="Bool"("DisabledEnum"=w1341) -> ()  [unwired: 2 in, 2 out]
      }
    }
    n1012 = property on="Next Patched Cell" class="Bool"("DisabledEnum"=w809) -> ()  [unwired: 2 in, 2 out]
    n1013 = property on="Previous Patched Cell" class="Bool"("DisabledEnum"=w803) -> ()  [unwired: 2 in, 2 out]
    n1014 = Array Size(array=w815) -> (size(s)=w818:i32)
    n1015 = Array Size(array=w774) -> (size(s)=w817:i32)
    n1016 = local read "Patched Cell Indicies"() -> (w801:i32[])
    n1017 = local read "Patched Cell Index"() -> (w802:dbl)
    n1018 = local write "unpatched+reserved"(w774) -> ()
    n1019 = Equal?(x=w818, y=w817) -> (x = y?=w816:bool)
    n1020 = Divide(x=w776, y=10.0) -> (x/y=w777:dbl[])
    n1021 = case shown="True" w816 {
      tunnel: [T56."Enabled" ("Disabled") T56."Disabled and Grayed Out" ("Disabled")] -> w813
      frame False {
      }
      frame True {
        # "The # of unpatched cells == the\n# of all cells selected..."
      }
    }
    n1022 = Index Array(array=w801, index=w802) -> (element=w773:i32)
    n1023 = local write "Current Manipulator Position [um]"(w777) -> ()
    n1024 = local write "Current Manipulator Position"(w776) -> ()
    n1025 = local write "Manip Being Calibrated Name"(w775) -> ()
    n1026 = local write "Patched Cell Value"(w773) -> ()
    n1027 = property on="Load Cells to Queue Button" class="Bool (strict)"("DisabledEnum"=w813) -> ()  [unwired: 2 in, 2 out]
    n1028 = Get Notifier Status(notifier=w832, error in (no error)=w834) -> (current notification=w835:bool, error out=w833:errorcluster)  [unwired: 3 out]
    n1029 = local write "Calibration Protocol"(w830) -> ()
    n1030 = property on="Restart Calibration Button" class="Bool (strict)"("Visible"=w828) -> ()  [unwired: 2 in, 2 out]
    n1031 = property on="Seek Backwards Calibration Button" class="Bool (strict)"("Visible"=w827) -> ()  [unwired: 2 in, 2 out]
    n1032 = property on="Accept Button" class="Bool (strict)"("Visible"=w827) -> ()  [unwired: 2 in, 2 out]
    n1033 = property on="Current Manipulator Position" class="Arr (strict)"("Visible"=TRUE) -> ()  [unwired: 2 in, 2 out]
    n1034 = property on="go to zero" class="Bool (strict)"("Visible"=TRUE) -> ()  [unwired: 2 in, 2 out]
  }
  n1035 = while {
    tunnel: w394 -> [w1371]
    tunnel: w398 -> [w1370]
    tunnel: [w1368] -> w395
    tunnel: w392 -> [_]
    tunnel: w270 -> [w1367]
    tunnel: w272 -> [w1366]
    stop <- w1369 stop-if-true
    # "Init Calibration Event Structure"
    n1036 = event shown="[2] \"Restart Calibration Button\": Mouse Up" {
      selector: _ -> [_ _ _ _ _ _ _ _ _ _ _ _ _ _ _ _ _]
      dyn-events: _ -> [_ _ _ _ _ _ _ _ _ _ _ _ _ _ _ _ _]
      timeout: 100 -> [_ _ _ _ _ _ _ _ _ _ _ _ _ _ _ _ _]
      tunnel: w1371 -> [w1376 _ _ _ _ _ _ _ _ _ _ _ _ _ _ _ _]
      tunnel: w1370 -> [w1375 _ _ _ _ _ _ _ _ _ _ _ _ _ _ _ _]
      tunnel: [w1374 _ _ _ _ _ _ _ _ _ _ _ _ _ _ _ _] -> w1369
      tunnel: [w1373 _ _ _ _ _ _ _ _ _ _ _ _ _ _ _ _] -> w1368
      tunnel: w1367 -> [_ _ _ _ _ _ _ _ _ _ _ _ _ w1412 _ _ _]
      tunnel: w1366 -> [_ _ _ _ _ _ _ _ _ _ _ _ _ w1411 _ _ _]
      event Timeout {
        n1037 = event-data() -> ()  [unwired: 1 in, 3 out]
        n1038 = Get Notifier Status(notifier=w1376, error in (no error)=w1375) -> (current notification=w1374:bool, error out=w1373:errorcluster)  [unwired: 3 out]
      }
      event "Calibration Button": Mouse Up {
        w1378 = T56."Enabled" ("Disabled")
        n1039 = event-data() -> ()  [unwired: 1 in, 8 out]
        n1040 = property on="Accept Button" class="Bool (strict)"("DisabledEnum"=w1378) -> ()  [unwired: 2 in, 2 out]
        n1041 = local write "Calibration Protocol"(T7."Select Manip" ("Calibration Protocol")) -> ()
        n1042 = property on="zero stage" class="Bool (strict)"("DisabledEnum"=w1378) -> ()  [unwired: 2 in, 2 out]
        n1043 = property on="current stage pos (steps)" class="Arr (strict)"("DisabledEnum"=w1378) -> ()  [unwired: 2 in, 2 out]
        n1044 = invoke on="Manip 3 Calibrated" class="Bool (strict)" method="Reinit To Default"() -> ()  [unwired: 3 in, 3 out]
        n1045 = invoke on="Manip 2 Calibrated" class="Bool (strict)" method="Reinit To Default"() -> ()  [unwired: 3 in, 3 out]
        n1046 = invoke on="Manip 1 Calibrated" class="Bool (strict)" method="Reinit To Default"() -> ()  [unwired: 3 in, 3 out]
        n1047 = invoke on="Manip 4 Calibrated" class="Bool (strict)" method="Reinit To Default"() -> ()  [unwired: 3 in, 3 out]
      }
      event "Restart Calibration Button": Mouse Up {
        n1048 = event-data() -> ()  [unwired: 1 in, 8 out]
        n1049 = local read "Calibrate:"() -> (w1381:T8)
        n1050 = case shown="\"manipulator 1\", Default" w1381 {
          tunnel: FALSE ("Visible") -> [w1383 w1384 w1385 w1386]
          frame "manipulator 1", Default {
            n1051 = local write "Manip 1 Calibrated"(w1383) -> ()
          }
          frame "manipulator 2" {
            n1052 = local write "Manip 2 Calibrated"(w1384) -> ()
          }
          frame "manipulator 3" {
            n1053 = local write "Manip 3 Calibrated"(w1385) -> ()
          }
          frame "manipulator 4" {
            n1054 = local write "Manip 4 Calibrated"(w1386) -> ()
          }
        }
        n1055 = invoke on="Restart Calibration Button" class="Bool (strict)" method="Reinit To Default"() -> ()  [unwired: 3 in, 3 out]
        n1056 = local write "Calibration Protocol"(T7."Select Manip" ("Calibration Protocol")) -> ()
        n1057 = property on="Accept Button" class="Bool (strict)"("DisabledEnum"=T56."Enabled" ("Disabled")) -> ()  [unwired: 2 in, 2 out]
      }
      event "Add More Cells Button": Mouse Up {
        n1058 = event-data() -> ()  [unwired: 1 in, 8 out]
        n1059 = invoke on="Add More Cells Button" class="Bool (strict)" method="Reinit To Default"() -> ()  [unwired: 3 in, 3 out]
        n1060 = local write "Calibration Protocol"(T7."Add Cells" ("Calibration Protocol")) -> ()
        n1061 = property on="Accept Button" class="Bool (strict)"("DisabledEnum"=T56."Enabled" ("Disabled")) -> ()  [unwired: 2 in, 2 out]
      }
      event "Load Cells to Queue Button": Value Change {
        n1062 = event-data() -> ("NewVal"=w1389:bool)  [unwired: 1 in, 5 out]
        n1063 = case shown="True" w1389 {
          frame False {
          }
          frame True {
            n1064 = local write "Calibration Protocol"(T7."Load Old Cells" ("Calibration Protocol")) -> ()
            n1065 = invoke on="Load Cells to Queue Button" class="Bool (strict)" method="Reinit To Default"() -> ()  [unwired: 3 in, 3 out]
            n1066 = property on="Accept Button" class="Bool (strict)"("DisabledEnum"=T56."Enabled" ("Disabled")) -> ()  [unwired: 2 in, 2 out]
          }
        }
      }
      event "Add this cell index into queue": Value Change {
        n1067 = event-data() -> ("NewVal"=w1392:bool)  [unwired: 1 in, 5 out]
        n1068 = case shown="True" w1392 {
          frame False {
          }
          frame True {
            n1069 = local read "unpatched cell indices"() -> (w1395:i32[])
            n1070 = local read "Patched Cell Value"() -> (w1393:dbl)
            n1071 = Build Array (concatenate)(w1395, w1393) -> (w1394:dbl[])
            n1072 = local write "unpatched cell indices"(w1394) -> ()
            n1073 = invoke on="Add this cell index into queue" class="Bool" method="Reinit To Default"() -> ()  [unwired: 3 in, 3 out]
          }
        }
      }
      event "Next Patched Cell": Mouse Up {
        n1074 = event-data() -> ()  [unwired: 1 in, 8 out]
        n1075 = local read "Patched Cell Index"() -> (w1397:dbl)
        n1076 = Increment(x=w1397) -> (x+1=w1396:dbl)
        n1077 = invoke on="Next Patched Cell" class="Bool" method="Reinit To Default"() -> ()  [unwired: 3 in, 3 out]
        n1078 = local write "Patched Cell Index"(w1396) -> ()
      }
      event "Previous Patched Cell": Mouse Up {
        n1079 = event-data() -> ()  [unwired: 1 in, 8 out]
        n1080 = local read "Patched Cell Index"() -> (w1399:dbl)
        n1081 = invoke on="Previous Patched Cell" class="Bool" method="Reinit To Default"() -> ()  [unwired: 3 in, 3 out]
        n1082 = Decrement(x=w1399) -> (x-1=w1398:dbl)
        n1083 = local write "Patched Cell Index"(w1398) -> ()
      }
      event "Skip Calibration Button": Mouse Up {
        n1084 = event-data() -> ()  [unwired: 1 in, 8 out]
        n1085 = local write "Calibration Protocol"(T7."Finish" ("Calibration Protocol")) -> ()
      }
      event "zero stage": Mouse Up {
        n1086 = event-data() -> ()  [unwired: 1 in, 8 out]
        n1087 = disable-structure shown="Disabled" {
          frame Disabled {
            n1088 = property on="zero stage" class="Bool (strict)"("DisabledEnum"=T56."Disabled and Grayed Out" ("Disabled")) -> ()  [unwired: 2 in, 2 out]
          }
          frame Enabled {
          }
        }
        n1089 = local write "Stage zeroed?"(TRUE ("Stage zeroed")) -> ()